vi "UHR-Fleezers Control (host) - 12.3.vi"() -> ()   [LabVIEW 2012] (continued)
        n1563 = event-data() -> ()  [unwired: 7 out]
        n1564 = xnode "Read/Write Control"("FPGA VI Reference In"=w2253, "error in"=w2252, "MCL count"="Update Count (MCL)") -> ("error out"=w2251:errorcluster)  [unwired: 1 out]
      }
      event "+ phase (MCL)", "- phase (MCL)": Value Change {
        n1565 = event-data() -> ()  [unwired: 7 out]
        n1566 = Or(x="- phase (MCL)", y="+ phase (MCL)") -> (x .or. y?=w2256:bool)
        n1567 = Negate(x="Phase adjust (MCL)") -> (-x=w2262:i16)
        n1568 = Select(t=w2262, s="+ phase (MCL)", f="Phase adjust (MCL)") -> (s? t:f=w2260:i16)
        n1569 = xnode "Read/Write Control"("FPGA VI Reference In"=w2264, "error in"=w2263, "Phase count adjustment (MCL)"=w2260) -> ("FPGA VI Reference Out"=w2257:T19, "error out"=w2258:errorcluster)
        n1570 = xnode "Read/Write Control"("FPGA VI Reference In"=w2257, "error in"=w2258, "+ phase (MCL)"=w2256) -> ("error out"=w2255:errorcluster)  [unwired: 1 out]
      }
      event "Abort AOD Scan": Value Change {
        n1571 = event-data() -> ()  [unwired: 7 out]
        n1572 = xnode "Read/Write Control"("FPGA VI Reference In"=w2268, "error in"=w2267, "Abort scan"="Abort AOD Scan") -> ("error out"=w2266:errorcluster)  [unwired: 1 out]
      }
      event "Continuous AOD Scanning": Value Change {
        n1573 = event-data() -> ()  [unwired: 7 out]
        n1574 = xnode "Read/Write Control"("FPGA VI Reference In"=w2272, "error in"=w2271, "Cont. Scan"="Continuous AOD Scanning") -> ("error out"=w2270:errorcluster)  [unwired: 1 out]
      }
      event "Index": Value Change {
        n1575 = event-data() -> ()  [unwired: 7 out]
        n1576 = call "Create new save file.vi"("Insert"="", "Ext"=".dat" ("string"), "Index In"="Index") -> ("Path Out"=→"Save file name":path, "Index Out"=w2273:dbl)
        "Save index" <- w2273
        n1577 = local write "Index"(w2273) -> ()
      }
      event "AO1", "AO2": Value Change {
        w2288 = 10.0 ("y")
        w2287 = 32767.0 ("y")
        n1578 = event-data() -> ()  [unwired: 7 out]
        n1579 = local read "AO2"() -> (w2286:dbl)
        n1580 = local read "AO1"() -> (w2283:dbl)
        n1581 = Multiply(x=w2283, y=w2287) -> (x*y=w2282:dbl)
        n1582 = Multiply(x=w2286, y=w2287) -> (x*y=w2285:dbl)
        n1583 = Divide(x=w2282, y=w2288) -> (x/y=w2281:dbl)
        n1584 = Divide(x=w2285, y=w2288) -> (x/y=w2284:dbl)
        n1585 = To Word Integer(number=w2281) -> (16bit integer=w2289:i16)
        n1586 = To Word Integer(number=w2284) -> (16bit integer=w2290:i16)
        n1587 = xnode "Read/Write Control"("FPGA VI Reference In"=w2280, "error in"=w2279, "AO1"=w2289, "AO2"=w2290) -> ("error out"=w2278:errorcluster)  [unwired: 1 out]
      }
      event "Inject Pump 1": Value Change {
        n1588 = event-data() -> ()  [unwired: 7 out]
        n1589 = local read "Use Harvard pumps\nfor beads (else Chemyx)"() -> (w2292:bool)
        n1590 = case shown="True" w2292 {
          tunnel: "Inject Pump 1" -> [w2296 w2334]
          tunnel: w2291 -> [_ w2335]
          frame False {
            n1591 = local read "Pump write delay (ms)"() -> (w2295:dbl)
            n1592 = local read "Chemyx Syringe Pump Serial Port"() -> (w2294:refnum<visa-resource-name>)
            n1593 = case shown="True" w2296 {
              tunnel: w2295 -> [w2302 w2316]
              tunnel: w2294 -> [w2299 w2315]
              frame False {
                n1594 = flat-sequence {
                  tunnel: w2299 -> [w2303]
                  tunnel: [w2303] -> w2300
                  tunnel: w2302 -> [_]
                  tunnel: [w2306] -> w2301
                  tunnel: w2300 -> [w2306]
                  tunnel: w2301 -> [w2307]
                  tunnel: [w2307] -> w2297
                  tunnel: [w2309] -> w2298
                  tunnel: w2297 -> [w2309]
                  tunnel: w2298 -> [w2311]
                  frame #0 {
                    n1595 = call "Write to pump.vi"("string"="enter pump1", "VISA resource name"=w2303) -> ()  [unwired: 1 out]
                  }
                  frame #1 {
                    n1596 = Wait (ms)(milliseconds to wait="Pump pause delay (ms)") -> ()  [unwired: 1 out]
                  }
                  frame #2 {
                    n1597 = call "Write to pump.vi"("string"="stop", "VISA resource name"=w2307) -> ()  [unwired: 1 out]
                  }
                  frame #3 {
                    n1598 = Wait (ms)(milliseconds to wait=u32 500) -> ()  [unwired: 1 out]
                  }
                  frame #4 {
                    n1599 = call "Write to pump.vi"("string"="stop", "VISA resource name"=w2311) -> ()  [unwired: 1 out]
                  }
                }
              }
              frame True {
                n1600 = flat-sequence {
                  tunnel: w2315 -> [w2325]
                  tunnel: w2316 -> [w2320]
                  tunnel: w2316 -> [w2327]
                  tunnel: w2315 -> [w2328]
                  tunnel: [w2328] -> w2313
                  tunnel: [w2330] -> w2314
                  tunnel: w2313 -> [w2330]
                  tunnel: w2314 -> [w2332]
                  frame #0 {
                    n1601 = local read "All Pump Parameters"() -> (w2319:T5)
                    n1602 = Unbundle By Name(w2319) -> ("Pump 1"=w2326:T29)
                    n1603 = call "Set pump parameters.vi"("Pump write delay (ms)"=w2320, "Volume (uL)"="Ch 1 Inject Volume (uL)", "Rate (uL/h)"="Ch 1 Inject Rate (ul/h)", "Units"=4.0, "Pump #"=1.0, "Pump Parameters In"=w2326, "VISA resource name"=w2325) -> ("Pump Parameters Out"=w2318:T29)  [unwired: 3 in]
                    n1604 = Bundle By Name(cluster=w2319, "Pump 1"=w2318) -> (w2317:T5)
                    n1605 = local write "All Pump Parameters"(w2317) -> ()
                  }
                  frame #1 {
                    n1606 = Wait (ms)(milliseconds to wait=w2327) -> ()  [unwired: 1 out]
                  }
                  frame #2 {
                    n1607 = call "Write to pump.vi"("string"="start", "VISA resource name"=w2328) -> ()  [unwired: 1 out]
                  }
                  frame #3 {
                    n1608 = Wait (ms)(milliseconds to wait=u32 500) -> ()  [unwired: 1 out]
                  }
                  frame #4 {
                    n1609 = call "Write to pump.vi"("string"="start", "VISA resource name"=w2332) -> ()  [unwired: 1 out]
                  }
                }
              }
            }
          }
          frame True {
            n1610 = case shown="False" w2334 {
              tunnel: w2335 -> [w2336 w2346]
              frame False {
                n1611 = flat-sequence {
                  tunnel: w2336 -> [w2338]
                  frame #0 {
                    n1612 = local write "Flushing P1"(FALSE ("Flushing P1")) -> ()
                    n1613 = Concatenate Strings("stop" ("string"), "\r") -> (w2340:string)
                    n1614 = VISA Write(VISA resource name=w2338, write buffer=w2340) -> ()  [unwired: 1 in, 3 out]
                  }
                  frame #1 {
                    n1615 = property on="Clear Volume P1" class="Bool (strict)"("Val(Sgnl)"=TRUE ("Value (Signaling)")) -> ()  [unwired: 2 in, 2 out]
                  }
                }
              }
              frame True {
                n1616 = local read "Normal Flow Rate (ul/h) P1"() -> (w2344:dbl)
                n1617 = Number To Decimal String(number=w2344) -> (decimal integer string=w2350:string)  [unwired: 1 in]
                n1618 = Concatenate Strings("irate  " ("string"), w2350, " u/h" ("string"), "\r") -> (w2348:string)
                n1619 = VISA Write(VISA resource name=w2346, write buffer=w2348) -> (VISA resource name out=w2345:refnum<visa-resource-name>)  [unwired: 1 in, 2 out]
                n1620 = Concatenate Strings("irun" ("string"), "\r") -> (w2352:string)
                n1621 = VISA Write(VISA resource name=w2345, write buffer=w2352) -> ()  [unwired: 1 in, 3 out]
              }
            }
          }
        }
      }
      event "Inject Pump 3": Value Change {
        n1622 = event-data() -> ()  [unwired: 7 out]
        n1623 = local read "Use Harvard pumps\nfor beads (else Chemyx)"() -> (w2355:bool)
        n1624 = case shown="True" w2355 {
          tunnel: "Inject Pump 3" -> [w2359 w2398]
          tunnel: w2354 -> [_ w2397]
          frame False {
            n1625 = local read "Pump write delay (ms)"() -> (w2358:dbl)
            n1626 = case shown="True" w2359 {
              tunnel: w2358 -> [w2365 w2379]
              tunnel: "Chemyx Syringe Pump Serial Port" -> [w2362 w2378]
              frame False {
                n1627 = flat-sequence {
                  tunnel: w2362 -> [w2366]
                  tunnel: [w2366] -> w2363
                  tunnel: w2365 -> [_]
                  tunnel: [w2369] -> w2364
                  tunnel: w2363 -> [w2369]
                  tunnel: w2364 -> [w2370]
                  tunnel: [w2370] -> w2360
                  tunnel: [w2372] -> w2361
                  tunnel: w2360 -> [w2372]
                  tunnel: w2361 -> [w2374]
                  frame #0 {
                    n1628 = call "Write to pump.vi"("string"="enter pump3", "VISA resource name"=w2366) -> ()  [unwired: 1 out]
                  }
                  frame #1 {
                    n1629 = local read "Pump pause delay (ms)"() -> (w2368:u32)
                    n1630 = Wait (ms)(milliseconds to wait=w2368) -> ()  [unwired: 1 out]
                  }
                  frame #2 {
                    n1631 = call "Write to pump.vi"("string"="stop", "VISA resource name"=w2370) -> ()  [unwired: 1 out]
                  }
                  frame #3 {
                    n1632 = Wait (ms)(milliseconds to wait=u32 0) -> ()  [unwired: 1 out]
                  }
                  frame #4 {
                    n1633 = call "Write to pump.vi"("string"="stop", "VISA resource name"=w2374) -> ()  [unwired: 1 out]
                  }
                }
              }
              frame True {
                n1634 = flat-sequence {
                  tunnel: w2378 -> [w2388]
                  tunnel: w2379 -> [w2383]
                  tunnel: w2379 -> [w2390]
                  tunnel: w2378 -> [w2391]
                  tunnel: [w2391] -> w2377
                  tunnel: [w2394] -> w2376
                  tunnel: w2377 -> [w2394]
                  tunnel: w2376 -> [w2395]
                  frame #0 {
                    n1635 = local read "All Pump Parameters"() -> (w2382:T5)
                    n1636 = Unbundle By Name(w2382) -> ("Pump 3"=w2389:T29)
                    n1637 = call "Set pump parameters.vi"("Pump write delay (ms)"=w2383, "Volume (uL)"="Ch 3 Inject Volume (uL)", "Rate (uL/h)"="Ch 3 Inject Rate (ul/h)", "Units"=4.0, "Pump #"=3.0, "Pump Parameters In"=w2389, "VISA resource name"=w2388) -> ("Pump Parameters Out"=w2381:T29)  [unwired: 3 in]
                    n1638 = Bundle By Name(cluster=w2382, "Pump 3"=w2381) -> (w2380:T5)
                    n1639 = local write "All Pump Parameters"(w2380) -> ()
                  }
                  frame #1 {
                    n1640 = Wait (ms)(milliseconds to wait=w2390) -> ()  [unwired: 1 out]
                  }
                  frame #2 {
                    n1641 = call "Write to pump.vi"("string"="start", "VISA resource name"=w2391) -> ()  [unwired: 1 out]
                  }
                  frame #3 {
                    n1642 = Wait (ms)(milliseconds to wait=u32 500) -> ()  [unwired: 1 out]
                  }
                  frame #4 {
                    n1643 = call "Write to pump.vi"("string"="start", "VISA resource name"=w2395) -> ()  [unwired: 1 out]
                  }
                }
              }
            }
          }
          frame True {
            n1644 = case shown="False" w2398 {
              tunnel: w2397 -> [w2399 w2406]
              frame False {
                n1645 = flat-sequence {
                  tunnel: w2399 -> [w2401]
                  frame #0 {
                    n1646 = local write "Flushing P3"(FALSE ("Flushing P3")) -> ()
                    n1647 = Concatenate Strings("stop" ("string"), "\r") -> (w2403:string)
                    n1648 = VISA Write(VISA resource name=w2401, write buffer=w2403) -> ()  [unwired: 1 in, 3 out]
                  }
                  frame #1 {
                    n1649 = property on="Clear Volume P3" class="Bool (strict)"("Val(Sgnl)"=TRUE ("Value (Signaling)")) -> ()  [unwired: 2 in, 2 out]
                  }
                }
              }
              frame True {
                n1650 = local read "Normal Flow Rate (ul/h) P3"() -> (w2407:dbl)
                n1651 = Number To Decimal String(number=w2407) -> (decimal integer string=w2413:string)  [unwired: 1 in]
                n1652 = Concatenate Strings("irate  " ("string"), w2413, " u/h" ("string"), "\r") -> (w2411:string)
                n1653 = VISA Write(VISA resource name=w2406, write buffer=w2411) -> (VISA resource name out=w2409:refnum<visa-resource-name>)  [unwired: 1 in, 2 out]
                n1654 = Concatenate Strings("irun" ("string"), "\r") -> (w2415:string)
                n1655 = VISA Write(VISA resource name=w2409, write buffer=w2415) -> ()  [unwired: 1 in, 3 out]
              }
            }
          }
        }
      }
      event "Inject Pump 2": Value Change {
        n1656 = event-data() -> ()  [unwired: 7 out]
        n1657 = local read "Pump write delay (ms)"() -> (w2419:dbl)
        n1658 = flat-sequence {
          tunnel: w2417 -> [w2432]
          tunnel: w2419 -> [w2428]
          tunnel: "Inject Pump 2" -> [_]
          tunnel: w2419 -> [w2434]
          tunnel: w2417 -> [w2435]
          frame #0 {
            n1659 = local read "All Pump Parameters"() -> (w2427:T5)
            n1660 = Multiply(x=60.0, y="Flush Center Ch Rate (ul/m)") -> (x*y=w2424:dbl)
            n1661 = Unbundle By Name(w2427) -> ("Pump 2"=w2433:T29)
            n1662 = call "Set pump parameters.vi"("Pump write delay (ms)"=w2428, "Volume (uL)"="Flush Center Ch Volume (uL)", "Rate (uL/h)"=w2424, "Units"=3.0, "Pump #"=2.0, "Pump Parameters In"=w2433, "VISA resource name"=w2432) -> ("Pump Parameters Out"=w2426:T29)  [unwired: 3 in]
            n1663 = Bundle By Name(cluster=w2427, "Pump 2"=w2426) -> (w2425:T5)
            n1664 = local write "All Pump Parameters"(w2425) -> ()
            n1665 = Add(x="Flush Center Ch Volume (uL)", y="Total Volume\nFlushed (uL)") -> (x+y=w2421:dbl)
            n1666 = local write "Total Volume\nFlushed (uL)"(w2421) -> ()
          }
          frame #1 {
            n1667 = Wait (ms)(milliseconds to wait=w2434) -> ()  [unwired: 1 out]
          }
          frame #2 {
            n1668 = call "Write to pump.vi"("string"="start", "VISA resource name"=w2435) -> ()  [unwired: 1 out]
          }
        }
        n1669 = local read "Chemyx Syringe Pump Serial Port"() -> (w2417:refnum<visa-resource-name>)
      }
      event "Sample Channel\nFlow": Value Change {
        n1670 = event-data() -> ()  [unwired: 7 out]
        n1671 = Select(t="irun" ("string"), s="Sample Channel\nFlow", f="stop" ("string")) -> (s? t:f=w2439:string)
        n1672 = Concatenate Strings(w2439, "\r") -> (w2442:string)
        n1673 = VISA Write(VISA resource name=w2437, write buffer=w2442) -> ()  [unwired: 1 in, 3 out]
      }
      event "Start Flow": Value Change {
        n1674 = event-data() -> ()  [unwired: 7 out]
        n1675 = local write "Sample Channel\nFlow"(TRUE ("Sample Channel\nFlow")) -> ()
        n1676 = local write "Start Flow"(FALSE ("Start Flow")) -> ()
        n1677 = Concatenate Strings("irun" ("string"), "\r") -> (w2448:string)
        n1678 = VISA Write(VISA resource name=w2444, write buffer=w2448) -> ()  [unwired: 1 in, 3 out]
      }
      event "Stop Flow": Value Change {
        w2450 = FALSE ("Stop Flow")
        n1679 = event-data() -> ()  [unwired: 7 out]
        n1680 = local write "Stop Flow"(w2450) -> ()
        n1681 = local write "Sample Channel\nFlow"(w2450) -> ()
        n1682 = Concatenate Strings("stop" ("string"), "\r") -> (w2453:string)
        n1683 = VISA Write(VISA resource name=w2451, write buffer=w2453) -> ()  [unwired: 1 in, 3 out]
      }
      event "Flow rate (uL/h)": Value Change {
        n1684 = event-data() -> ()  [unwired: 7 out]
        n1685 = Number To Decimal String(number="Flow rate (uL/h)") -> (decimal integer string=w2460:string)  [unwired: 1 in]
        n1686 = Concatenate Strings("irate  " ("string"), w2460, " u/h" ("string"), "\r") -> (w2459:string)
        n1687 = VISA Write(VISA resource name=w2456, write buffer=w2459) -> ()  [unwired: 1 in, 3 out]
      }
      event "Flush Sample": Value Change {
        n1688 = event-data() -> ()  [unwired: 7 out]
        n1689 = flat-sequence {
          tunnel: w2465 -> [w2493]
          tunnel: [w2473] -> w2464
          tunnel: [w2467] -> w2462
          tunnel: w2464 -> [w2497]
          tunnel: [w2497] -> w2463
          tunnel: w2462 -> [w2496]
          tunnel: w2463 -> [w2502]
          frame #0 {
            # "set paramaters (rate, volume) for flush, clear volume"
            n1690 = Number To Decimal String(number="Flush rate (uL/m)") -> (decimal integer string=w2489:string)  [unwired: 1 in]
            n1691 = Concatenate Strings("irate  " ("string"), w2489, " u/m" ("string"), "\r") -> (w2491:string)
            n1692 = VISA Write(VISA resource name=w2493, write buffer=w2491) -> (VISA resource name out=w2487:refnum<visa-resource-name>)  [unwired: 1 in, 2 out]
            n1693 = Reciprocal(x="Flush rate (uL/m)") -> (1/x=w2470:dbl)
            n1694 = Number To Decimal String(number="Volume (uL)") -> (decimal integer string=w2478:string)  [unwired: 1 in]
            n1695 = Multiply(x="Volume (uL)", y=w2470) -> (x*y=w2469:dbl)
            n1696 = Concatenate Strings("tvolume  " ("string"), w2478, " u" ("string"), "\r") -> (w2476:string)
            n1697 = Multiply(x=w2469, y=60000.0) -> (x*y=w2467:dbl)
            n1698 = VISA Write(VISA resource name=w2487, write buffer=w2476) -> (VISA resource name out=w2475:refnum<visa-resource-name>)  [unwired: 1 in, 2 out]
            n1699 = Concatenate Strings("cvolume" ("string"), "\r") -> (w2474:string)
            n1700 = VISA Write(VISA resource name=w2475, write buffer=w2474) -> (VISA resource name out=w2485:refnum<visa-resource-name>)  [unwired: 1 in, 2 out]
            n1701 = Concatenate Strings("irun" ("string"), "\r") -> (w2483:string)
            n1702 = VISA Write(VISA resource name=w2485, write buffer=w2483) -> (VISA resource name out=w2473:refnum<visa-resource-name>)  [unwired: 1 in, 2 out]
          }
          frame #1 {
            # "Have to wait until\nflow is done to reset\nrate"
            n1703 = Add(x=w2496, y=100.0) -> (x+y=w2495:dbl)
            n1704 = Wait (ms)(milliseconds to wait=w2495) -> ()  [unwired: 1 out]
          }
          frame #2 {
            # "reset flow rate to usual flow rate"
            n1705 = local read "Flow rate (uL/h)"() -> (w2508:dbl)
            n1706 = Number To Decimal String(number=w2508) -> (decimal integer string=w2506:string)  [unwired: 1 in]
            n1707 = Concatenate Strings("irate  " ("string"), w2506, " u/h" ("string"), "\r") -> (w2504:string)
            n1708 = VISA Write(VISA resource name=w2502, write buffer=w2504) -> (VISA resource name out=w2498:refnum<visa-resource-name>)  [unwired: 1 in, 2 out]
            n1709 = Concatenate Strings("cvolume" ("string"), "\r") -> (w2499:string)
            n1710 = VISA Write(VISA resource name=w2498, write buffer=w2499) -> ()  [unwired: 1 in, 3 out]
          }
        }
      }
      event "Flush Pump 3": Value Change {
        n1711 = event-data() -> ()  [unwired: 7 out]
        n1712 = flat-sequence {
          tunnel: w2509 -> [w2512]
          frame #0 {
            # "set paramaters (rate, volume) for flush, clear volume"
            n1713 = Number To Decimal String(number="Flush rate (uL/m) P3") -> (decimal integer string=w2534:string)  [unwired: 1 in]
            n1714 = local write "Inject Pump 3"(TRUE ("Inject Pump 3")) -> ()
            n1715 = Concatenate Strings("irate  " ("string"), w2534, " u/m" ("string"), "\r") -> (w2536:string)
            n1716 = VISA Write(VISA resource name=w2512, write buffer=w2536) -> (VISA resource name out=w2532:refnum<visa-resource-name>)  [unwired: 1 in, 2 out]
            n1717 = Reciprocal(x="Flush rate (uL/m) P3") -> (1/x=w2516:dbl)
            n1718 = Number To Decimal String(number="Volume (uL) P3") -> (decimal integer string=w2523:string)  [unwired: 1 in]
            n1719 = Multiply(x="Volume (uL) P3", y=w2516) -> (x*y=w2515:dbl)
            n1720 = Concatenate Strings("tvolume  " ("string"), w2523, " u" ("string"), "\r") -> (w2521:string)
            n1721 = Multiply(x=w2515, y=60.0) -> (x*y=→"HP3 Flush Time (s)":dbl)
            n1722 = VISA Write(VISA resource name=w2532, write buffer=w2521) -> (VISA resource name out=w2520:refnum<visa-resource-name>)  [unwired: 1 in, 2 out]
            n1723 = Concatenate Strings("cvolume" ("string"), "\r") -> (w2519:string)
            n1724 = VISA Write(VISA resource name=w2520, write buffer=w2519) -> (VISA resource name out=w2530:refnum<visa-resource-name>)  [unwired: 1 in, 2 out]
            n1725 = Concatenate Strings("irun" ("string"), "\r") -> (w2528:string)
            n1726 = VISA Write(VISA resource name=w2530, write buffer=w2528) -> ()  [unwired: 1 in, 3 out]
          }
          frame #1 {
            "Flushing P3" <- TRUE ("Flushing P3")
          }
        }
      }
      event "Flush Pump 1": Value Change {
        n1727 = event-data() -> ()  [unwired: 7 out]
        n1728 = flat-sequence {
          tunnel: [w2550] -> w2540
          tunnel: w2539 -> [w2543]
          tunnel: w2540 -> [_]
          frame #0 {
            # "set paramaters (rate, volume) for flush, clear volume"
            n1729 = local write "Inject Pump 1"(TRUE ("Inject Pump 1")) -> ()
            n1730 = Number To Decimal String(number="Flush rate (uL/m) P1") -> (decimal integer string=w2566:string)  [unwired: 1 in]
            n1731 = Concatenate Strings("irate  " ("string"), w2566, " u/m" ("string"), "\r") -> (w2568:string)
            n1732 = VISA Write(VISA resource name=w2543, write buffer=w2568) -> (VISA resource name out=w2564:refnum<visa-resource-name>)  [unwired: 1 in, 2 out]
            n1733 = Reciprocal(x="Flush rate (uL/m) P1") -> (1/x=w2547:dbl)
            n1734 = Number To Decimal String(number="Volume (uL) P1") -> (decimal integer string=w2555:string)  [unwired: 1 in]
            n1735 = Multiply(x="Volume (uL) P1", y=w2547) -> (x*y=w2546:dbl)
            n1736 = Concatenate Strings("tvolume  " ("string"), w2555, " u" ("string"), "\r") -> (w2553:string)
            n1737 = Multiply(x=w2546, y=60.0) -> (x*y=→"HP1 Flush Time (s)":dbl)
            n1738 = VISA Write(VISA resource name=w2564, write buffer=w2553) -> (VISA resource name out=w2552:refnum<visa-resource-name>)  [unwired: 1 in, 2 out]
            n1739 = Concatenate Strings("cvolume" ("string"), "\r") -> (w2551:string)
            n1740 = VISA Write(VISA resource name=w2552, write buffer=w2551) -> (VISA resource name out=w2562:refnum<visa-resource-name>)  [unwired: 1 in, 2 out]
            n1741 = Concatenate Strings("irun" ("string"), "\r") -> (w2560:string)
            n1742 = VISA Write(VISA resource name=w2562, write buffer=w2560) -> (VISA resource name out=w2550:refnum<visa-resource-name>)  [unwired: 1 in, 2 out]
          }
          frame #1 {
            "Flushing P1" <- TRUE ("Flushing P3")
          }
        }
      }
      event "Clear Volume": Value Change {
        n1743 = event-data() -> ()  [unwired: 7 out]
        n1744 = Concatenate Strings("cvolume" ("string"), "\r") -> (w2572:string)
        n1745 = VISA Write(VISA resource name=w2571, write buffer=w2572) -> ()  [unwired: 1 in, 3 out]
      }
      event "Clear Volume P3": Value Change {
        n1746 = event-data() -> ()  [unwired: 7 out]
        n1747 = Concatenate Strings("cvolume" ("string"), "\r") -> (w2578:string)
        n1748 = VISA Write(VISA resource name=w2577, write buffer=w2578) -> ()  [unwired: 1 in, 3 out]
        n1749 = local write "Clear Volume P3"(FALSE ("Clear Volume P3")) -> ()
      }
      event "Clear Volume P1": Value Change {
        n1750 = event-data() -> ()  [unwired: 7 out]
        n1751 = Concatenate Strings("cvolume" ("string"), "\r") -> (w2583:string)
        n1752 = local write "Clear Volume P1"(FALSE ("Clear Volume P1")) -> ()
        n1753 = VISA Write(VISA resource name=w2582, write buffer=w2583) -> ()  [unwired: 1 in, 3 out]
      }
      event "Display On P3": Value Change {
        n1754 = event-data() -> ()  [unwired: 7 out]
        n1755 = Select(t="dim 100", s="Display On P3", f="dim 0") -> (s? t:f=w2589:string)
        n1756 = Concatenate Strings(w2589, "\r") -> (w2591:string)
        n1757 = VISA Write(VISA resource name=w2586, write buffer=w2591) -> ()  [unwired: 1 in, 3 out]
      }
      event "Display On P1": Value Change {
        n1758 = event-data() -> ()  [unwired: 7 out]
        n1759 = Select(t="dim 100", s="Display On P1", f="dim 0") -> (s? t:f=w2596:string)
        n1760 = Concatenate Strings(w2596, "\r") -> (w2598:string)
        n1761 = VISA Write(VISA resource name=w2593, write buffer=w2598) -> ()  [unwired: 1 in, 3 out]
      }
      event "Retract Pump 3": Value Change {
        n1762 = event-data() -> ()  [unwired: 7 out]
        n1763 = local write "Retract Pump 3"(FALSE ("Retract Pump 3")) -> ()
        n1764 = case shown="True" "Retract Pump 3" {
          tunnel: w2600 -> [_ w2603]
          frame False {
          }
          frame True {
            n1765 = Number To Decimal String(number="Retract Rate (uL/m)") -> (decimal integer string=w2621:string)  [unwired: 1 in]
            n1766 = Concatenate Strings("wrate  " ("string"), w2621, " u/m" ("string"), "\r") -> (w2623:string)
            n1767 = VISA Write(VISA resource name=w2603, write buffer=w2623) -> (VISA resource name out=w2614:refnum<visa-resource-name>)  [unwired: 1 in, 2 out]
            n1768 = Number To Decimal String(number="Retract Vol 3 (uL)") -> (decimal integer string=w2616:string)  [unwired: 1 in]
            n1769 = Concatenate Strings("tvolume  " ("string"), w2616, " u" ("string"), "\r") -> (w2613:string)
            n1770 = VISA Write(VISA resource name=w2614, write buffer=w2613) -> (VISA resource name out=w2609:refnum<visa-resource-name>)  [unwired: 1 in, 2 out]
            n1771 = Concatenate Strings("cvolume" ("string"), "\r") -> (w2610:string)
            n1772 = VISA Write(VISA resource name=w2609, write buffer=w2610) -> (VISA resource name out=w2604:refnum<visa-resource-name>)  [unwired: 1 in, 2 out]
            n1773 = Concatenate Strings("wrun" ("string"), "\r") -> (w2605:string)
            n1774 = VISA Write(VISA resource name=w2604, write buffer=w2605) -> ()  [unwired: 1 in, 3 out]
          }
        }
      }
      event "Retract Pump 1": Value Change {
        n1775 = event-data() -> ()  [unwired: 7 out]
        n1776 = local write "Retract Pump 1"(FALSE ("Retract Pump 1")) -> ()
        n1777 = case shown="True" "Retract Pump 1" {
          tunnel: w2625 -> [_ w2630]
          frame False {
          }
          frame True {
            n1778 = local read "Retract Rate (uL/m)"() -> (w2628:dbl)
            n1779 = Number To Decimal String(number=w2628) -> (decimal integer string=w2646:string)  [unwired: 1 in]
            n1780 = Concatenate Strings("wrate  " ("string"), w2646, " u/m" ("string"), "\r") -> (w2648:string)
            n1781 = VISA Write(VISA resource name=w2630, write buffer=w2648) -> (VISA resource name out=w2640:refnum<visa-resource-name>)  [unwired: 1 in, 2 out]
            n1782 = Number To Decimal String(number="Retract Vol 1 (uL)") -> (decimal integer string=w2642:string)  [unwired: 1 in]
            n1783 = Concatenate Strings("tvolume  " ("string"), w2642, " u" ("string"), "\r") -> (w2639:string)
            n1784 = VISA Write(VISA resource name=w2640, write buffer=w2639) -> (VISA resource name out=w2636:refnum<visa-resource-name>)  [unwired: 1 in, 2 out]
            n1785 = Concatenate Strings("cvolume" ("string"), "\r") -> (w2637:string)
            n1786 = VISA Write(VISA resource name=w2636, write buffer=w2637) -> (VISA resource name out=w2631:refnum<visa-resource-name>)  [unwired: 1 in, 2 out]
            n1787 = Concatenate Strings("wrun" ("string"), "\r") -> (w2632:string)
            n1788 = VISA Write(VISA resource name=w2631, write buffer=w2632) -> ()  [unwired: 1 in, 3 out]
          }
        }
      }
      event "Flip Green Filter": Value Change {
        n1789 = event-data() -> ()  [unwired: 7 out]
        n1790 = Not(x="Flip Green Filter") -> (.not. x?=w2650:bool)
        n1791 = local write "Flip Green Filter"(w2650) -> ()
        n1792 = flat-sequence {
          tunnel: w2658 -> [w2663]
          tunnel: w2657 -> [w2662]
          tunnel: [w2660] -> w2655
          tunnel: [w2659] -> w2654
          tunnel: [w2665] -> w2653
          tunnel: w2655 -> [w2665]
          tunnel: [w2664] -> w2652
          tunnel: w2654 -> [w2664]
          tunnel: w2653 -> [w2669]
          tunnel: w2652 -> [w2668]
          tunnel: [w2667] -> w2656
          frame #0 {
            n1793 = xnode "Read/Write Control"("FPGA VI Reference In"=w2663, "error in"=w2662, "Green Filter Flipper"=TRUE) -> ("FPGA VI Reference Out"=w2660:T19, "error out"=w2659:errorcluster)
          }
          frame #1 {
            n1794 = Wait (ms)(milliseconds to wait=u32 100) -> ()  [unwired: 1 out]
          }
          frame #2 {
            n1795 = xnode "Read/Write Control"("FPGA VI Reference In"=w2669, "error in"=w2668, "Green Filter Flipper"=FALSE) -> ("error out"=w2667:errorcluster)  [unwired: 1 out]
          }
        }
      }
      event "Pump 1 contents", "Pump 3 contents": Value Change {
        n1796 = event-data() -> ()  [unwired: 7 out]
        n1797 = local read "Pump 1 contents"() -> (→"Pump 1 cont disp":string)
        n1798 = local read "Pump 3 contents"() -> (→"Pump 3 cont disp":string)
      }
      event "Reset Trap Pos. FB": Value Change {
        n1799 = event-data() -> ()  [unwired: 7 out]
        n1800 = xnode "Read/Write Control"("FPGA VI Reference In"=w2675, "error in"=w2674, "Trap Pos. FB Reset"="Reset Trap Pos. FB") -> ()  [unwired: 2 out]
      }
      event "Rem fb disp offset": Value Change {
        n1801 = event-data() -> ()  [unwired: 7 out]
        n1802 = local write "Rem fb disp offset"(FALSE ("Rem fb disp offset")) -> ()
        n1803 = local read "Mean T1 Position (nm)"() -> (w2677:dbl)
        n1804 = local read "FB Trap Pos Offset"() -> (w2678:dbl)
        n1805 = Subtract(x=w2678, y=w2677) -> (x-y=w2676:dbl)
        n1806 = local write "FB Trap Pos Offset"(w2676) -> ()
      }
      event "Threshold (nm)": Value Change {
        n1807 = event-data() -> ()  [unwired: 7 out]
        n1808 = flat-sequence {
          tunnel: w2682 -> [w2690]
          tunnel: w2681 -> [w2689]
          tunnel: [w2683] -> w2680
          tunnel: w2680 -> [w2696]
          frame #0 {
            n1809 = xnode "Read/Write Control"("FPGA VI Reference In"=w2690, "error in"=w2689) -> ("FPGA VI Reference Out"=w2686:T19, "error out"=w2685:errorcluster, "FPGA TTrig Thresh"=w2687:i64)
            n1810 = local read "Threshold stored (nm)"() -> (w2695:dbl)
            n1811 = local read "Threshold (nm)"() -> (w2683:dbl)
            n1812 = local read "AOM X Cal (nm/MHz)"() -> (w2693:dbl)
            n1813 = Subtract(x=w2683, y=w2695) -> (x-y=w2694:dbl)
            n1814 = Divide(x=w2694, y=w2693) -> (x/y=w2691:dbl)
            n1815 = call "IR AOM freq to word.vi"("Frequency In (MHz)"=w2691) -> ("Frequency Word Out (double)"=w2692:dbl)
            n1816 = To Quad Integer(1:w2692) -> (0:w2688:i64)
            n1817 = Add(x=w2687, y=w2688) -> (x+y=w2684:i64)
            n1818 = xnode "Read/Write Control"("FPGA VI Reference In"=w2686, "error in"=w2685, "FPGA TTrig Thresh"=w2684) -> ()  [unwired: 2 out]
          }
          frame #1 {
            "Threshold stored (nm)" <- w2696
          }
        }
      }
      event "FB Trig Integrate": Value Change {
        n1819 = event-data() -> ()  [unwired: 7 out]
        n1820 = local read "FB Trig Integrate"() -> (w2698:u32)
        n1821 = xnode "Read/Write Control"("FPGA VI Reference In"=w2700, "error in"=w2699, "FB Trig Integrate"=w2698) -> ("error out"=w2697:errorcluster)  [unwired: 1 out]
      }
      event "11": Value Change {
        n1822 = event-data() -> ()  [unwired: 7 out]
        n1823 = local read "11"() -> (w2701:bool)
        n1824 = case shown="True" w2701 {
          frame False {
          }
          frame True {
            n1825 = local read "Messages"() -> (w2703:string)
            n1826 = call "Update messages.vi"("Message to add"="You kicked it up to 11!", "Old message string"=w2703) -> ("New message string"=w2704:string)
            n1827 = call <vilib>:"Beep.vi"() -> ()  [unwired: 12 in]
            n1828 = local write "Messages"(w2704) -> ()
          }
        }
      }
      event "Trap Pos. FB ON": Value Change {
        n1829 = event-data() -> ()  [unwired: 7 out]
        n1830 = xnode "Read/Write Control"("FPGA VI Reference In"=w2707, "error in"=w2706, "Force feedback"="Trap Pos. FB ON") -> ()  [unwired: 2 out]
      }
      event "Remove Action Offset": Value Change {
        n1831 = event-data() -> ()  [unwired: 7 out]
        n1832 = local write "Remove Action Offset"(FALSE ("Remove Action Offset")) -> ()
        n1833 = local read "Trap Pos. FB Mult Factor"() -> (w2712:i64)
        n1834 = local read "Trap Pos FB Action"() -> (w2710:i64)
        n1835 = local read "Trap Pos. FB Offset Factor"() -> (w2708:i64)
        n1836 = Multiply(x=w2712, y=w2710) -> (x*y=w2711:i64)
        n1837 = Add(x=w2711, y=w2708) -> (x+y=w2709:i64)
        n1838 = local write "Trap Pos. FB Offset Factor"(w2709) -> ()
        n1839 = xnode "Read/Write Control"("FPGA VI Reference In"=w2715, "error in"=w2714, "Trap Pos. FB Offset Factor"=w2709) -> ()  [unwired: 2 out]
      }
      event "Remove Unwinding Offset": Value Change {
        n1840 = event-data() -> ()  [unwired: 7 out]
        n1841 = local write "Remove Unwinding Offset"(FALSE ("Remove Action Offset")) -> ()
        n1842 = local read "Trap Pos. FB Mult Factor"() -> (w2727:i64)
        n1843 = local read "Trap Pos FB Action"() -> (w2725:i64)
        n1844 = local read "Trap Pos. FB Offset Factor"() -> (w2724:i64)
        n1845 = Multiply(x=w2727, y=w2725) -> (x*y=w2726:i64)
        n1846 = local read "Trap Pos. FB Mult Factor"() -> (w2723:i64)
        n1847 = Add(x=w2726, y=w2724) -> (x+y=w2717:i64)
        n1848 = Multiply(x=32768, y="factor") -> (x*y=w2720:dbl)
        n1849 = Multiply(x=w2720, y=w2723) -> (x*y=w2722:dbl)
        n1850 = Subtract(x=w2717, y=w2722) -> (x-y=w2721:dbl)
        n1851 = To Quad Integer(1:w2721) -> (0:w2716:i64)
        n1852 = xnode "Read/Write Control"("FPGA VI Reference In"=w2730, "error in"=w2729, "Trap Pos. FB Offset Factor"=w2716) -> ()  [unwired: 2 out]
        n1853 = local write "Trap Pos. FB Offset Factor"(w2716) -> ()
      }
      event "Trap Pos. FB Range", "Trap Pos. FB Gains", "Trap Pos. FB Mult Factor", "Trap Pos. FB Offset Factor", "Trap Pos FB Negate Action", "Trap Pos FB Monitor\nT1 or T2", "Differential FB?", "Negate Diff?": Value Change {
        n1854 = event-data() -> ()  [unwired: 7 out]
        n1855 = Unbundle By Name("Trap Pos. FB Gains") -> ("proportional gain (Kc)"=w2733:fxp<+/-,16,8>, "integral gain (Kc*Ts/Ti)"=w2732:fxp<+/-,16,8>, "derivative gain (Kc*Td/Ts)"=w2731:fxp<+/-,16,8>)
        n1856 = local read "Negate Diff?"() -> (w2738:bool)
        n1857 = Unbundle By Name("Trap Pos. FB Range") -> ("output high"=w2736:fxp<+/-,16,1>, "output low"=w2735:fxp<+/-,16,1>)
        n1858 = xnode "Read/Write Control"("FPGA VI Reference In"=w2746, "error in"=w2745, "FB2 output high"=w2736, "FB2 output low"=w2735, "P2"=w2733, "I2"=w2732, "D2"=w2731, "Trap Pos. FB Mult Factor"="Trap Pos. FB Mult Factor", "Trap Pos. FB Offset Factor"="Trap Pos. FB Offset Factor", "Trap Pos FB Negate Action"="Trap Pos FB Negate Action", "Trap Pos FB Monitor T1 or T2"="Trap Pos FB Monitor\nT1 or T2", "AI1 X Scale"="Trap Pos. AI1 X Pre-scale", "Negate Diff?"=w2738, "Diff FB Measurement?"="Differential FB?") -> ()  [unwired: 2 out]
      }
      event "Trap Pos FB SP", "Trap Pos FB SP 2", "Use SP 2": Value Change {
        n1859 = event-data() -> ()  [unwired: 7 out]
        n1860 = Select(t="Trap Pos FB SP 2", s="Use SP 2", f="Trap Pos FB SP") -> (s? t:f=w2747:fxp<+/-,16,1>)
        n1861 = xnode "Read/Write Control"("FPGA VI Reference In"=w2752, "error in"=w2751, "Trap Pos. FB SP"=w2747) -> ()  [unwired: 2 out]
      }
      event "Offset SP2 from SP1": Value Change {
        n1862 = event-data() -> ()  [unwired: 7 out]
        n1863 = local read "Trap Pos FB SP"() -> (w2755:fxp<+/-,16,1>)
        n1864 = Add(x=w2755, y="SP2 Offset") -> (x+y=w2753:fxp<+/-,16,1>)
        n1865 = property on="Trap Pos FB SP 2" class="DigNum (strict)"("Val(Sgnl)"=w2753) -> ()  [unwired: 2 in, 2 out]
        n1866 = local write "Offset SP2 from SP1"(FALSE ("Offset SP2 from SP1")) -> ()
      }
      event "Set Reading to\nSetpoint": Value Change {
        # "This is the actual PID input signal"
        n1867 = event-data() -> ()  [unwired: 7 out]
        n1868 = local write "Set Reading to\nSetpoint"(FALSE ("Set SP to Reading")) -> ()
        n1869 = xnode "Read/Write Control"("FPGA VI Reference In"=w2761, "error in"=w2760) -> ("FPGA VI Reference Out"=w2759:T19, "error out"=w2758:errorcluster, "Trap Pos FB Int-Norm Signal"=w2757:fxp<+/-,16,1>)
        n1870 = local read "Differential FB?"() -> (w2762:bool)
        n1871 = case shown="False" w2762 {
          tunnel: [w2767 w2774] -> w2764
          tunnel: w2757 -> [w2765 w2774]
          frame False {
            n1872 = local read "Trap Pos FB Monitor\nT1 or T2"() -> (w2770:bool)
            n1873 = local read "Trap X AI1 (DMA)"() -> (w2773:T13)
            n1874 = Unbundle By Name(w2773) -> ("Set 1"=w2772:fxp<+/-,16,1>, "Set 2"=w2771:fxp<+/-,16,1>)
            n1875 = Select(t=w2772, s=w2770, f=w2771) -> (s? t:f=w2769:fxp<+/-,16,1>)
            n1876 = Not(x="Set SP Using...") -> (.not. x?=w2766:bool)
            n1877 = Select(t=w2765, s=w2766, f=w2769) -> (s? t:f=w2767:fxp<+/-,16,1>)
          }
          frame True {
          }
        }
        n1878 = xnode "Read/Write Control"("FPGA VI Reference In"=w2759, "error in"=w2758, "Trap Pos. FB SP"=w2764) -> ()  [unwired: 2 out]
        n1879 = local write "Trap Pos FB SP"(w2764) -> ()
      }
      event "Trap Pos. FB Out Scale 2^n": Value Change {
        n1880 = event-data() -> ()  [unwired: 7 out]
        n1881 = Scale By Power Of 2(n="Trap Pos. FB Out Scale 2^n", x=ext 1.0) -> (x*2^n=w2775:ext)
        n1882 = property on="Trap Pos. FB Mult Factor" class="DigNum (strict)"("Val(Sgnl)"=w2775) -> ()  [unwired: 2 in, 2 out]
      }
      event "Trap Pos FB Int Count": Value Change {
        n1883 = event-data() -> ()  [unwired: 7 out]
        n1884 = xnode "Read/Write Control"("FPGA VI Reference In"=w2780, "error in"=w2779, "Trap Pos FB Int Count"="Trap Pos FB Int Count") -> ()  [unwired: 2 out]
      }
      event "Trap pos": Value Change {
        n1885 = event-data() -> ()  [unwired: 7 out]
        n1886 = case shown="True" "Trap pos" {
          frame False {
            n1887 = property on="Trap Delta Graph" class="WFGraph (strict)"("Visible"=TRUE) -> ()  [unwired: 2 in, 2 out]
            n1888 = property on="Saved trap pos" class="WFGraph (strict)"("Visible"=FALSE) -> ()  [unwired: 2 in, 2 out]
          }
          frame True {
            n1889 = property on="Saved trap pos" class="WFGraph (strict)"("Visible"=TRUE) -> ()  [unwired: 2 in, 2 out]
            n1890 = property on="Trap Delta Graph" class="WFGraph (strict)"("Visible"=FALSE) -> ()  [unwired: 2 in, 2 out]
          }
        }
      }
    }
    "error out 2" <- w1590
    n1891 = node-c288() -> ()  [unwired: 2 out]
  }
  n1892 = timed-loop "Mouse control: trap position (AOM deflection), set confocal spot from image" {
    tunnel: [w2787] -> w202
    tunnel: w8 -> [w2786]
    timing: w124 -> [_]
    timing-out: [_] -> w123
    stop <- w2787 stop-if-true
    n1893 = node-c288() -> ()  [unwired: 2 out]
    n1894 = event shown="[0] \"Pane\": Mouse Down" {
      selector: _ -> [_ _]
      dyn-events: _ -> [_ _]
      timeout: _ -> [_ _]
      tunnel: w2786 -> [w2790 _]
      event Mouse Down {
        n1895 = event-data() -> ("Time"=w2792:u32, "Coords"=w2791:T7, "Button"=w2793:u16)  [unwired: 6 out]
        n1896 = case shown="1" w2793 {
          tunnel: w2792 -> [_ _ w2899]
          tunnel: w2791 -> [_ w2830 w2897]
          tunnel: w2790 -> [_ _ w2895]
          frame 0, Default {
          }
          frame 1 {
            n1897 = property on="APD 2" class="ImageControl"() -> ("Displayed Image Position"=w2800:cluster{"Left":i32, "Top":i32})  [unwired: 2 in, 2 out]
            n1898 = property on="APD 1" class="ImageControl"() -> ("Displayed Image Position"=w2829:cluster{"Left":i32, "Top":i32})  [unwired: 2 in, 2 out]
            n1899 = property on="Detection Laser X" class="ImageControl"() -> ("Displayed Image Position"=w2826:cluster{"Left":i32, "Top":i32})  [unwired: 2 in, 2 out]
            n1900 = property on="Detection Laser Y" class="ImageControl"() -> ("Displayed Image Position"=w2825:cluster{"Left":i32, "Top":i32})  [unwired: 2 in, 2 out]
            n1901 = property on="APD 2" class="ImageControl"() -> ("Displayed Image Size"=w2799:cluster{"Width":u32, "Height":u32})  [unwired: 2 in, 2 out]
            n1902 = property on="APD 1" class="ImageControl"() -> ("Displayed Image Size"=w2827:cluster{"Width":u32, "Height":u32})  [unwired: 2 in, 2 out]
            n1903 = property on="Detection Laser X" class="ImageControl"() -> ("Displayed Image Size"=w2828:cluster{"Width":u32, "Height":u32})  [unwired: 2 in, 2 out]
            n1904 = property on="Detection Laser Y" class="ImageControl"() -> ("Displayed Image Size"=w2824:cluster{"Width":u32, "Height":u32})  [unwired: 2 in, 2 out]
            n1905 = Unbundle By Name(w2799) -> ("Width"=w2796:u32, "Height"=w2795:u32)
            n1906 = Unbundle By Name(w2800) -> ("Left"=w2798:i32, "Top"=w2797:i32)
            n1907 = Unbundle By Name(w2827) -> ("Width"=w2821:u32, "Height"=w2820:u32)
            n1908 = Unbundle By Name(w2828) -> ("Width"=w2817:u32, "Height"=w2816:u32)
            n1909 = Unbundle By Name(w2824) -> ("Width"=w2813:u32, "Height"=w2812:u32)
            n1910 = Unbundle By Name(w2829) -> ("Left"=w2823:i32, "Top"=w2822:i32)
            n1911 = Unbundle By Name(w2826) -> ("Left"=w2819:i32, "Top"=w2818:i32)
            n1912 = Unbundle By Name(w2825) -> ("Left"=w2815:i32, "Top"=w2814:i32)
            n1913 = Bundle("Left"=w2798, "Top"=w2797, "Width"=w2796, "Height"=w2795) -> (w2794:T30)  [unwired: 1 in]
            n1914 = Bundle("Left"=w2823, "Top"=w2822, "Width"=w2821, "Height"=w2820) -> (w2811:T30)  [unwired: 1 in]
            n1915 = Bundle("Left"=w2819, "Top"=w2818, "Width"=w2817, "Height"=w2816) -> (w2810:T30)  [unwired: 1 in]
            n1916 = Bundle("Left"=w2815, "Top"=w2814, "Width"=w2813, "Height"=w2812) -> (w2809:T30)  [unwired: 1 in]
            n1917 = Build Cluster Array(w2794, w2811, w2810, w2809) -> (w2808:T31)
            n1918 = for {
              tunnel: w2830 -> [w2841]
              tunnel: w2808 -> [w2842] mode=indexing
              shift-right: [w2839] -> w2806
              shift-left: TRUE -> [w2840]
              shift-right: [w2838] -> w2804
              shift-left: _ -> [w2834]
              shift-right: [w2837] -> w2803
              shift-left: _ -> [w2833]
              shift-right: [w2836] -> w2802
              shift-left: _ -> [w2832]
              shift-right: [w2835] -> w2801
              shift-left: _ -> [w2831]
              n1919 = case shown="True" w2840 {
                selector: w2840 -> [w2847 _]
                tunnel: w2842 -> [_ w2856]
                tunnel: w2841 -> [_ w2854]
                tunnel: [w2847 w2852] -> w2839
                tunnel: [w2846 w2851] -> w2838
                tunnel: [w2845 w2850] -> w2837
                tunnel: [w2844 w2849] -> w2836
                tunnel: [w2843 w2848] -> w2835
                tunnel: w2834 -> [w2846 _]
                tunnel: w2833 -> [w2845 _]
                tunnel: w2832 -> [w2844 _]
                tunnel: w2831 -> [w2843 _]
                frame False {
                }
                frame True {
                  n1920 = Unbundle(w2856) -> (w2855:T30)
                  n1921 = call "isclickinwindow.vi"("Image Param"=w2855, "Point32"=w2854) -> ("4 Y"=w2848:i32, "3 Height"=w2849:i32, "2 X"=w2850:i32, "1 Width"=w2851:i32, "In image?"=w2853:bool)  [unwired: 1 in]
                  n1922 = Not(x=w2853) -> (.not. x?=w2852:bool)
                }
              }
            }
            n1923 = Not(x=w2806) -> (.not. x?=w2805:bool)
            n1924 = case shown="True" w2805 {
              tunnel: w2803 -> [_ w2870]
              tunnel: w2801 -> [_ w2869]
              tunnel: w2804 -> [_ w2868]
              tunnel: w2802 -> [_ w2867]
              frame False {
              }
              frame True {
                w2857 = FALSE ("Get Point")
                n1925 = local read "Scan lines (y)"() -> (w2872:u64)
                n1926 = disable-structure shown="Disabled" {
                  frame Disabled {
                  }
                  frame Enabled {
                  }
                }
                n1927 = local read "Actual MCL Inc (V)"() -> (w2866:dbl)
                n1928 = local read "Scan steps (MCL)"() -> (w2871:u64)
                n1929 = Divide "Y Pix/step"(x=w2867, y=w2872) -> (x/y=w2879:dbl)
                n1930 = Divide "Y V/pix"(x=w2866, y=w2879) -> (x/y=w2878:dbl)
                n1931 = Divide "Y half step offset"(x=w2866, y=2.0) -> (x/y=w2880:dbl)
                n1932 = Divide "X pix/step"(x=w2868, y=w2871) -> (x/y=w2877:dbl)
                n1933 = Negate(x=w2880) -> (-x=w2881:dbl)
                n1934 = local read "Initial Y"() -> (w2887:dbl)
                n1935 = Multiply(x=w2869, y=w2878) -> (x*y=w2888:dbl)
                n1936 = Divide "X half step offset"(x=w2866, y=2.0) -> (x/y=w2874:dbl)
                n1937 = Divide "X V/pix"(x=w2866, y=w2877) -> (x/y=w2876:dbl)
                n1938 = Multiply(x=w2866, y=w2871) -> (x*y=w2883:dbl)
                n1939 = Compound Arithmetic op=ADD(w2881, w2888, w2887) -> (w2858:dbl)
                "Pointer Y (V)" <- w2858
                n1940 = Multiply(x=w2876, y=w2870) -> (x*y=w2885:dbl)
                n1941 = Negate(x=w2874) -> (-x=w2873:dbl)
                n1942 = local read "Initial X"() -> (w2886:dbl)
                n1943 = Negate(x=w2885) -> (-x=w2884:dbl)
                n1944 = Compound Arithmetic op=ADD(w2873, w2883, w2886, w2884) -> (w2859:dbl)
                "Pointer X (V)" <- w2859
                n1945 = case shown="True" "Set High F Confocal Spot (X-Y)" {
                  tunnel: w2859 -> [_ w2889]
                  tunnel: w2858 -> [_ w2890]
                  frame False {
                  }
                  frame True {
                    "Confocal Y 2 (V)" <- w2890
                    "Confocal X 2 (V)" <- w2889
                  }
                }
                n1946 = Or(x="Set X Only", y="Set Confocal Spot (X-Y)") -> (x .or. y?=w2862:bool)
                n1947 = Or(x="Set Confocal Spot (X-Y)", y="Set Y Only") -> (x .or. y?=w2861:bool)
                n1948 = case shown="True" w2862 {
                  tunnel: w2859 -> [_ w2891]
                  frame False {
                  }
                  frame True {
                    n1949 = property on="AO2" class="Slide (strict)"("Val(Sgnl)"=w2891) -> ()  [unwired: 2 in, 2 out]
                    "Confocal X 1 (V)" <- w2891
                  }
                }
                n1950 = case shown="True" w2861 {
                  tunnel: w2858 -> [_ w2892]
                  frame False {
                  }
                  frame True {
                    n1951 = property on="AO1" class="Slide (strict)"("Val(Sgnl)"=w2892) -> ()  [unwired: 2 in, 2 out]
                    "Confocal Y 1 (V)" <- w2892
                  }
                }
                n1952 = local write "Set High F Confocal Spot (X-Y)"(w2857) -> ()
                n1953 = local write "Set Confocal Spot (X-Y)"(w2857) -> ()
                n1954 = local write "Set X Only"(w2857) -> ()
                n1955 = local write "Set Y Only"(w2857) -> ()
              }
            }
          }
          frame 3 {
            n1956 = local read "BD 2 Frequency 1 (MHz)"() -> (w2893:dbl)
            n1957 = local read "BD 1 Frequency 1 (MHz)"() -> (w2894:dbl)
            n1958 = local write "Manipulating Trap"(TRUE ("Manipulating Trap")) -> ()
            n1959 = local write "Coords"(T7 {"Horizontal"=0, "Vertical"=0} ("Coords")) -> ()
            n1960 = while {
              tunnel: w2899 -> [w2904]
              tunnel: w2897 -> [w2903]
              tunnel: w2895 -> [w2902]
              tunnel: w2894 -> [w2901]
              tunnel: w2893 -> [w2900]
              stop <- w2905 stop-if-true
              n1961 = event shown="[0] \"Pane\": Mouse Move" {
                selector: _ -> [_ _]
                dyn-events: _ -> [_ _]
                timeout: _ -> [_ _]
                tunnel: ["Force Manip Abort" w2969] -> w2905
                tunnel: w2904 -> [w2912 _]
                tunnel: w2903 -> [w2910 _]
                tunnel: w2902 -> [w2909 _]
                tunnel: w2901 -> [w2908 _]
                tunnel: w2900 -> [w2907 _]
                event Mouse Move {
                  n1962 = event-data() -> ("Time"=w2913:u32, "Coords"=w2914:T7)  [unwired: 3 out]
                  n1963 = Less?(x=w2913, y=w2912) -> (x < y?=w2911:bool)
                  n1964 = case "Makes sure old motion events prior to mouse click aren't used" shown="False" w2911 {
                    tunnel: w2914 -> [w2956 _]
                    tunnel: w2910 -> [w2957 _]
                    tunnel: w2909 -> [w2934 _]
                    tunnel: w2908 -> [w2930 _]
                    tunnel: w2907 -> [w2929 _]
                    frame False {
                      n1965 = Subtract(x=w2956, y=w2957) -> (x-y=w2955:T7)
                      "Coords" <- w2955
                      n1966 = local read "Y RF Frequency Limits (MHz)"() -> (w2915:T16)
                      n1967 = To Double Precision Float(number=w2955) -> (double precision float=w2954:cluster{"Horizontal":dbl, "Vertical":dbl})
                      n1968 = Multiply(x=cluster{"Horizontal":dbl, "Vertical":dbl} {"Horizontal"=-1.0, "Vertical"=1.0}, y="Manipulation Scaling") -> (x*y=w2950:cluster{"Horizontal":dbl, "Vertical":dbl})
                      n1969 = local read "X RF Frequency Limits (MHz)"() -> (w2916:T16)
                      n1970 = Multiply(x=w2954, y=w2950) -> (x*y=w2952:cluster{"Horizontal":dbl, "Vertical":dbl})
                      n1971 = Unbundle By Name(w2952) -> ("Horizontal"=w2947:dbl, "Vertical"=w2951:dbl)
                      n1972 = Unbundle By Name(w2915) -> ("Maximum"=w2918:dbl, "Minimum"=w2917:dbl)
                      n1973 = Boolean To (0,1)(Boolean="Manip. X?") -> (0, 1=w2945:i16)
                      n1974 = Boolean To (0,1)(Boolean="Manip. Y?") -> (0, 1=w2942:i16)
                      n1975 = local read "BD 1 Frequency 2 (MHz)"() -> (w2932:dbl)
                      n1976 = Multiply(x=w2951, y=w2942) -> (x*y=w2944:dbl)
                      n1977 = Multiply(x=w2945, y=w2947) -> (x*y=w2948:dbl)
                      n1978 = local read "BD 2 Frequency 2 (MHz)"() -> (w2931:dbl)
                      n1979 = Unbundle By Name(w2916) -> ("Maximum"=w2920:dbl, "Minimum"=w2919:dbl)
                      n1980 = Add(x=w2929, y=w2944) -> (x+y=w2922:dbl)
                      n1981 = Add(x=w2930, y=w2948) -> (x+y=w2924:dbl)
                      n1982 = In Range and Coerce(upper limit=w2920, x=w2924, lower limit=w2919) -> (coerced(x)=w2923:dbl)  [unwired: 1 out]
                      n1983 = In Range and Coerce(upper limit=w2918, x=w2922, lower limit=w2917) -> (coerced(x)=w2921:dbl)  [unwired: 1 out]
                      n1984 = Subtract(x=w2923, y=w2932) -> (x-y=w2941:dbl)
                      n1985 = Subtract(x=w2921, y=w2931) -> (x-y=w2940:dbl)